vi "Controle_Manip_Main_GUI_WorkingBackup_211222.vi"() -> ()   [LabVIEW 2019] (continued)
            n3621 = call "Shutter.vi"("KCube Shutter Device Reference 2"=w4454, "Shutter Ctrls 2"=w4455, "Shutter on?"=w4453) -> ()
          }
          event "Shutter Mode": Value Change {
            n3622 = event-data() -> ()  [unwired: 1 in, 6 out]
            n3623 = local read "KCube Shutter On?"() -> (w4456:bool)
            n3624 = case shown="True" w4456 {
              frame False {
              }
              frame True {
                # "1 Active == Laser on / Shutter off\n2 Inactive == Laser off / Shutter on\n\nThere are 4 operating modes for shutter:\n1 Manual\n2 Single Toggle\n3 Automatic Toggle\n4 Triggered"
                n3625 = local read "KCube Shutter Device Reference"() -> (w4458:refnum<k24>)
                n3626 = local read "Shutter Mode"() -> (w4457:i32)
                n3627 = invoke class="KCubeSolenoid" method="SetOperatingMode"(reference=w4458, "mode"=w4457) -> ()  [unwired: 2 in, 4 out]
              }
            }
          }
          event "Stop Everything & Quit?": Value Change {
            # "Stop program"
            n3628 = event-data() -> ("NewVal"=w4459:bool)  [unwired: 1 in, 5 out]
            "NewVal" <- w4459
          }
          event "TEC Output", "TEC Temperature", "Laser on? Control": Mouse Down; "Laser Diode Current Set": Value Change {
            # "Laser diode control"
            n3629 = event-data() -> ("CtlRef"=w4461:refnum<vi>)  [unwired: 1 in, 3 out]
            n3630 = local read "Laser Comm On?"() -> (w4460:bool)
            n3631 = case shown="True" w4460 {
              tunnel: w4461 -> [_ w4471]
              frame False {
              }
              frame True {
                n3632 = local read "Photodiode error out"() -> (w4470:errorcluster)
                n3633 = local read "Diode Driver Error"() -> (w4466:errorcluster)
                n3634 = local read "Photodiode handle out"() -> (w4469:refnum<visa-resource-name>)
                n3635 = property class="Ctl"(reference=w4471) -> ("Label.Text"=w4462:string)  [unwired: 1 in, 2 out]
                n3636 = local read "DDE"() -> (w4464:refnum<visa-resource-name>)
                n3637 = case shown="\"Laser on? Control\"" w4462 {
                  tunnel: w4464 -> [w4477 w4488 w4524 w4561 w4594]
                  tunnel: [w4476 w4487 w4523 w4563 w4594] -> w4467
                  tunnel: w4469 -> [w4474 w4483 w4522 w4564 w4593]
                  tunnel: w4470 -> [w4475 w4482 w4521 w4565 w4592]
                  tunnel: [w4474 w4479 w4520 w4564 w4593] -> w4468
                  tunnel: [w4475 w4484 w4519 w4565 w4592] -> w4463
                  tunnel: [w4473 w4481 w4518 w4562 w4591] -> w4465
                  tunnel: w4466 -> [w4472 w4480 w4517 w4560 w4591]
                  frame "TEC Temperature" {
                    n3638 = call <instrlib>:"TL4000 Measure Temperature.vi"("error in (no error)"=w4472, "instrument handle"=w4477) -> ("error out"=w4473:errorcluster, "Temperature"=w4478:dbl, "instrument handle out"=w4476:refnum<visa-resource-name>)  [unwired: 7 in]
                    n3639 = local write "TEC Temperature"(w4478) -> ()
                  }
                  frame "Laser on? Control" {
                    n3640 = flat-sequence {
                      tunnel: w4488 -> [w4496]
                      tunnel: [w4495] -> w4486
                      tunnel: [w4494] -> w4485
                      tunnel: w4480 -> [w4489]
                      tunnel: [w4507] -> w4487
                      tunnel: [w4508] -> w4481
                      tunnel: w4486 -> [w4508]
                      tunnel: w4485 -> [w4507]
                      tunnel: [w4506] -> w4479
                      tunnel: [w4505] -> w4484
                      tunnel: w4483 -> [w4504]
                      tunnel: w4482 -> [w4503]
                      frame #0 {
                        n3641 = call <instrlib>:"TL4000 Get LD Output State.vi"("error in (no error)"=w4489, "instrument handle"=w4496) -> ("error out"=w4491:errorcluster, "LD Output"=w4493:bool, "instrument handle out"=w4492:refnum<visa-resource-name>)  [unwired: 7 in]
                        n3642 = Not(x=w4493) -> (.not. x?=w4490:bool)
                        n3643 = case shown="True" w4490 {
                          selector: w4490 -> [w4498 w4499]
                          frame False {
                            n3644 = Not(x=w4498) -> (.not. x?=w4497:bool)
                            n3645 = property on="TEC Output" class="Bool (strict)"("Visible"=w4497) -> ()  [unwired: 2 in, 2 out]
                          }
                          frame True {
                            n3646 = property on="TEC Output" class="Bool (strict)"("Visible"=w4499) -> ()  [unwired: 2 in, 2 out]
                          }
                        }
                        n3647 = property on="Laser Diode Current Set" class="Slide (strict)"("Visible"=w4490) -> ()  [unwired: 2 in, 2 out]
                        n3648 = property on="Laser Safety" class="Ring (strict)"("Visible"=w4490) -> ()  [unwired: 2 in, 2 out]
                        n3649 = local write "Laser on?"(w4490) -> ()
                        n3650 = call <instrlib>:"TL4000 Switch LD Output.vi"("error in (no error)"=w4491, "LD Output (Off)"=w4490, "instrument handle"=w4492) -> ("error out"=w4495:errorcluster, "instrument handle out"=w4494:refnum<visa-resource-name>)  [unwired: 7 in]
                      }
                      frame #1 {
                        n3651 = local read "PM16-120 On?"() -> (w4500:bool)
                        n3652 = case shown="True" w4500 {
                          tunnel: [w4509 w4516] -> w4506
                          tunnel: [w4510 w4515] -> w4505
                          tunnel: w4504 -> [w4509 w4514]
                          tunnel: w4503 -> [w4510 w4513]
                          tunnel: [0.0 ("Power") w4512] -> w4502
                          frame False {
                          }
                          frame True {
                            n3653 = call <instrlib>:"TLPM Measure Power.vi"("error in (no error)"=w4513, "instrument handle"=w4514) -> ("error out"=w4515:errorcluster, "Power"=w4512:dbl, "instrument handle out"=w4516:refnum<visa-resource-name>)  [unwired: 7 in]
                          }
                        }
                        n3654 = local write "Excitation Power (uW)"(w4502) -> ()
                        n3655 = property on="Excitation Source" class="Enum (strict)"("Val(Sgnl)"=enum16{"P", "CW", "SK"}."CW" ("Value (Signaling)")) -> ()  [unwired: 2 in, 2 out]
                      }
                    }
                  }
                  frame "Laser Diode Current Set" {
                    n3656 = stacked-sequence {
                      seq-local: [w4529 _ _ _] -> [_ _ w4549 _]
                      seq-local: [w4528 _ _ _] -> [_ _ w4548 _]
                      tunnel: w4524 -> [w4533 _ _ _]
                      tunnel: w4517 -> [w4525 _ _ _]
                      tunnel: [_ _ w4549 _] -> w4523
                      tunnel: [_ _ w4548 _] -> w4518
                      tunnel: w4522 -> [_ _ w4547 _]
                      tunnel: w4521 -> [_ _ w4546 _]
                      tunnel: [_ _ w4545 _] -> w4520
                      tunnel: [_ _ w4544 _] -> w4519
                      frame #0 {
                        n3657 = local read "Laser Diode Current Set"() -> (w4526:dbl)
                        n3658 = call <instrlib>:"TL4000 Get Laser Diode Current Setpoint.vi"("error in (no error)"=w4525, "instrument handle"=w4533) -> ("error out"=w4530:errorcluster, "Laser Diode Current Setpoint"=w4532:dbl, "instrument handle out"=w4531:refnum<visa-resource-name>)  [unwired: 7 in]
                        n3659 = Not Equal?(x=w4526, y=w4532) -> (x != y?=w4527:bool)
                        n3660 = case shown="True" w4527 {
                          tunnel: w4531 -> [w4535 w4540]
                          tunnel: w4530 -> [w4534 w4539]
                          tunnel: [w4535 w4538] -> w4529
                          tunnel: [w4534 w4537] -> w4528
                          tunnel: w4526 -> [_ w4536]
                          frame False {
                          }
                          frame True {
                            n3661 = call <instrlib>:"TL4000 Set Laser Diode Current Setpoint.vi"("error in (no error)"=w4539, "Laser Diode Current Setpoint (0.0)"=w4536, "instrument handle"=w4540) -> ("error out"=w4537:errorcluster, "instrument handle out"=w4538:refnum<visa-resource-name>)  [unwired: 7 in]
                          }
                        }
                      }
                      frame #1 {
                        n3662 = Wait (ms)(milliseconds to wait=u32 50) -> ()  [unwired: 1 out]
                      }
                      frame #2 {
                        n3663 = local read "PM16-120 On?"() -> (w4542:bool)
                        n3664 = case shown="True" w4542 {
                          tunnel: w4547 -> [w4552 w4557]
                          tunnel: w4546 -> [w4551 w4556]
                          tunnel: [w4552 w4555] -> w4545
                          tunnel: [w4551 w4554] -> w4544
                          tunnel: [0.0 ("Power") w4553] -> w4543
                          frame False {
                          }
                          frame True {
                            n3665 = call <instrlib>:"TLPM Measure Power.vi"("error in (no error)"=w4556, "instrument handle"=w4557) -> ("error out"=w4554:errorcluster, "Power"=w4553:dbl, "instrument handle out"=w4555:refnum<visa-resource-name>)  [unwired: 7 in]
                          }
                        }
                        n3666 = local write "Excitation Power (uW)"(w4543) -> ()
                      }
                      frame #3 {
                        n3667 = local write "Background taken?"(FALSE ("Background taken?")) -> ()
                      }
                    }
                  }
                  frame "TEC Output" {
                    n3668 = local read "TEC Output"() -> (w4559:bool)
                    n3669 = call <instrlib>:"TL4000 Switch TEC Output.vi"("error in (no error)"=w4560, "TEC Output (Off)"=w4559, "instrument handle"=w4561) -> ("error out"=w4566:errorcluster, "instrument handle out"=w4567:refnum<visa-resource-name>)  [unwired: 7 in]
                    n3670 = case shown="True" w4559 {
                      tunnel: w4567 -> [w4569 w4576]
                      tunnel: w4566 -> [w4568 w4575]
                      tunnel: [w4569 w4572] -> w4563
                      tunnel: [w4568 w4571] -> w4562
                      frame False {
                      }
                      frame True {
                        n3671 = while {
                          tunnel: w4576 -> [w4590]
                          tunnel: [w4582] -> w4573
                          tunnel: w4575 -> [w4589]
                          tunnel: [w4583] -> w4574
                          stop <- w4577 stop-if-true
                          n3672 = call <instrlib>:"TL4000 Measure Temperature.vi"("error in (no error)"=w4589, "instrument handle"=w4590) -> ("error out"=w4583:errorcluster, "Temperature"=w4580:dbl, "instrument handle out"=w4582:refnum<visa-resource-name>)  [unwired: 7 in]
                          n3673 = Wait (ms)(milliseconds to wait=u32 250) -> ()  [unwired: 1 out]
                          n3674 = local write "TEC Temperature"(w4580) -> ()
                          n3675 = Subtract(x=w4580, y=25.0) -> (x-y=w4587:dbl)
                          n3676 = Absolute Value(x=w4587) -> (abs(x)=w4586:dbl)
                          n3677 = Equal?(x=w4580, y=0.0) -> (x = y?=w4578:bool)
                          n3678 = Less?(x=w4586, y=0.01) -> (x < y?=w4581:bool)
                          n3679 = Or(x=w4581, y=w4578) -> (x .or. y?=w4577:bool)
                        }
                        n3680 = call <instrlib>:"TL4000 Measure Temperature.vi"("error in (no error)"=w4574, "instrument handle"=w4573) -> ("error out"=w4571:errorcluster, "Temperature"=w4570:dbl, "instrument handle out"=w4572:refnum<visa-resource-name>)  [unwired: 7 in]
                        n3681 = local write "TEC Temperature"(w4570) -> ()
                      }
                    }
                    n3682 = property on="Laser on? Control" class="Bool (strict)"("Visible"=w4559) -> ()  [unwired: 2 in, 2 out]
                  }
                  frame Default {
                  }
                }
                "Diode Driver Error out" <- w4465
                n3683 = local write "Photodiode error out"(w4463) -> ()
                n3684 = local write "Photodiode handle out"(w4468) -> ()
                n3685 = local write "Diode Driver COM"(w4467) -> ()
              }
            }
          }
          event "Fit?": Mouse Down {
            n3686 = event-data() -> ()  [unwired: 1 in, 8 out]
            n3687 = property on="CCD 1D Spectrum Main" class="XYGraph (strict)"() -> ("Value"=w4599:cluster{dbl[], dbl[]})  [unwired: 2 in, 2 out]
            n3688 = local read "BackgroundSpec"() -> (w4595:dbl[])
            n3689 = Unbundle(w4599) -> (w4598:dbl[], w4596:dbl[])
            n3690 = call "subVI_FitLorentzien.vi"("Background Spec"=w4595, "X"=w4598, "Y"=w4596) -> ("best fit parameters"=→"best fit parameters":dbl[])  [unwired: 1 in, 3 out]
          }
          event "Temperature (K)": Mouse Down {
            n3691 = event-data() -> ()  [unwired: 1 in, 8 out]
            n3692 = local read "Cryostation On?"() -> (w4600:bool)
            n3693 = case shown="True" w4600 {
              frame False {
              }
              frame True {
                w4602 = 10.0 ("y")
                n3694 = local read "Cryostation ID"() -> (w4612:refnum<k5>)
                n3695 = call "GetCryoInfo.vi"("connection ID"=w4612) -> ("User Stability"=w4607:dbl, "User Temp"=w4608:dbl, "connection ID out"=w4606:refnum<k5>, "Sample Stability"=w4609:dbl, "Sample Temp"=w4605:dbl, "Platform Stability"=w4610:dbl, "Platform Temp"=w4611:dbl)  [unwired: 4 in]
                n3696 = local write "Cryo Platform Temp"(w4611) -> ()
                n3697 = Multiply(x=w4605, y=w4602) -> (x*y=w4604:dbl)
                n3698 = local write "Cryo Sample Stability"(w4609) -> ()
                n3699 = local write "Cryostation ID"(w4606) -> ()
                n3700 = local write "Cryo User Stability"(w4607) -> ()
                n3701 = local write "Cryo Sample Temp"(w4605) -> ()
                n3702 = local write "Cryo Platform Stability"(w4610) -> ()
                n3703 = local write "Cryo User Temp"(w4608) -> ()
                n3704 = Round To Nearest(number=w4604) -> (nearest integer value=w4603:dbl)
                n3705 = Divide(x=w4603, y=w4602) -> (x/y=w4601:dbl)
                n3706 = local write "Temperature (K)"(w4601) -> ()
              }
            }
          }
          event "Voltage Output?": Value Change {
            w4617 = u8 2 items=["1", "2", "3"] ("axis")
            w4618 = u8 1 items=["1", "2", "3"] ("axis")
            w4619 = u8 0 items=["1", "2", "3"] ("axis")
            n3707 = event-data() -> ("NewVal"=w4613:bool)  [unwired: 1 in, 5 out]
            n3708 = local read "Att DeviceHandle"() -> (w4628:u64)
            n3709 = local read "Att Error"() -> (w4626:errorcluster)
            n3710 = local read "ourDLL"() -> (w4616:path)
            n3711 = call "ANC350v4_SetAxisOutput.vi"("deviceHandle"=w4628, "Path to *.DLL"=w4616, "axis"=w4619, "enable"=w4613, "autoDisable"=TRUE, "error in"=w4626) -> ("deviceHandle"=w4624:u64, "error ANC350v4_setAxisOutput"=w4625:errorcluster)  [unwired: 7 in, 1 out]
            n3712 = call "ANC350v4_SetAxisOutput.vi"("deviceHandle"=w4624, "Path to *.DLL"=w4616, "axis"=w4618, "enable"=w4613, "autoDisable"=TRUE, "error in"=w4625) -> ("deviceHandle"=w4623:u64, "error ANC350v4_setAxisOutput"=w4622:errorcluster)  [unwired: 7 in, 1 out]
            n3713 = call "ANC350v4_SetAxisOutput.vi"("deviceHandle"=w4623, "Path to *.DLL"=w4616, "axis"=w4617, "enable"=w4613, "autoDisable"=TRUE, "error in"=w4622) -> ("deviceHandle"=w4615:u64, "error ANC350v4_setAxisOutput"=w4614:errorcluster)  [unwired: 7 in, 1 out]
            n3714 = local write "Att Error"(w4614) -> ()
            n3715 = local write "Att DeviceHandle"(w4615) -> ()
          }
          event Timeout {
            # "Use timeout case to send data to globals"
            n3716 = event-data() -> ()  [unwired: 1 in, 3 out]
          }
        }
      }
      n3717 = while {
        stop <- w696 stop-if-true
        # "Separate loop for \"measurements\" requiring simultaneous optimisation of experimental parameters: continuous modes"
        n3718 = event shown="[2] \"Acquire PD\": Mouse Down" {
          selector: _ -> [_ _ _]
          dyn-events: _ -> [_ _ _]
          timeout: 500 -> [_ _ _]
          event Timeout {
            n3719 = event-data() -> ()  [unwired: 1 in, 3 out]
          }
          event "Fast Acq Continuous": Mouse Down {
            n3720 = event-data() -> ()  [unwired: 1 in, 8 out]
            n3721 = local read "Acq Mode"() -> (w697:T3)
            n3722 = case shown="\"Spectrum\", Default" w697 {
              frame "Image" {
              }
              frame "APD 1" {
              }
              frame "Spectrum", Default {
                n3723 = stacked-sequence {
                  frame #0 {
                    # "prep stuff"
                    n3724 = property on="Experiment Graph Controls" class="TabCtl (strict)"("Value"=T25."Spectrum" ("Experiment Graph Controls")) -> ()  [unwired: 2 in, 2 out]
                  }
                  frame #1 {
                    # "open shutter once"
                    n3725 = control-ref of="Shutter Ctrls"() -> (w704:refnum<vi>)
                    n3726 = local read "KCube Shutter On?"() -> (w701:bool)
                    n3727 = local read "Acq Mode"() -> (w702:T3)
                    n3728 = control-ref of="KCube Shutter Device Reference"() -> (w703:refnum<vi>)
                    n3729 = call "Shutter.vi"("KCube Shutter Device Reference 2"=w703, "Shutter Ctrls 2"=w704, "Shutter on?"=w701) -> ()
                    n3730 = case shown="\"Spectrum\", Default" w702 {
                      frame "Spectrum", Default {
                        n3731 = property on="CCD 1D Spectrum Main" class="XYGraph (strict)"("Visible"=TRUE) -> ()  [unwired: 2 in, 2 out]
                        n3732 = property on="CCD 2D Image Main" class="IntGraph (strict)"("Visible"=FALSE) -> ()  [unwired: 2 in, 2 out]
                      }
                      frame "Image" {
                        n3733 = property on="CCD 1D Spectrum Main" class="XYGraph (strict)"("Visible"=FALSE) -> ()  [unwired: 2 in, 2 out]
                        n3734 = property on="CCD 2D Image Main" class="IntGraph (strict)"("Visible"=TRUE) -> ()  [unwired: 2 in, 2 out]
                      }
                    }
                    n3735 = control-ref of="MasterStop"() -> (w700:refnum<vi>)
                    n3736 = property class="Bool (strict)"(reference=w700, "Visible"=TRUE) -> ()  [unwired: 1 in, 2 out]
                  }
                  frame #2 {
                    # "acquire 1000 spectra"
                    n3737 = for {
                      N: 1000 -> [_]
                      stop <- w724 stop-if-true
                      n3738 = local read "CCD ROI"() -> (w719:T20)
                      n3739 = local read "LightField Automation out"() -> (w723:refnum<class "LightField Automation.lvclass">)
                      n3740 = local read "Acq Mode"() -> (w726:T3)
                      n3741 = local read "LightField Automation error out"() -> (w720:errorcluster)
                      n3742 = local read "Accumulations"() -> (w727:dbl)
                      n3743 = control-ref of="MasterStop"() -> (w710:refnum<vi>)
                      n3744 = local read "BackgroundSpec"() -> (w712:dbl[])
                      n3745 = local read "Excitation Power (uW)"() -> (w715:dbl)
                      n3746 = call "LFA_Capture.vi"("error in (no error)"=w720, "Frames"=w727, "LightField Automation in"=w723) -> ("error out"=w721:errorcluster, "Data"=w725:T26, "LightField Automation out"=w722:refnum<class "LightField Automation.lvclass">)  [unwired: 6 in]
                      n3747 = case shown="\"Spectrum\", Default" w726 {
                        selector: w726 -> [w735 w741]
                        tunnel: w725 -> [w736 w743]
                        tunnel: w719 -> [w732 w738]
                        tunnel: [w728 w737] -> w716
                        frame "Spectrum", Default {
                          n3748 = local read "Wavelength calibration"() -> (w730:dbl[])
                          n3749 = Divide(x=1239.842, y=w730) -> (x/y=w729:dbl[])
                          n3750 = call "PrepareData4Graph.vi"("Wavelength nm"=w729, "DataLF"=w736, "CCD ROI"=w732, "AcqMode"=w735, "Data type"=T30."Spectre") -> ("Spectrum"=w734:cluster{"Array 2":dbl[], "Array":dbl[]}, "PLInt out"=w728:dbl[])  [unwired: 2 in, 2 out]
                          n3751 = local write "CCD 1D Spectrum Main"(w734) -> ()
                        }
                        frame "Image" {
                          n3752 = local read "Wavelength calibration"() -> (w742:dbl[])
                          n3753 = call "PrepareData4Graph.vi"("Wavelength nm"=w742, "DataLF"=w743, "CCD ROI"=w738, "AcqMode"=w741, "Data type"=T30."Spectre") -> ("Intensity Graph"=w740:dbl[][], "PLInt out"=w737:dbl[])  [unwired: 2 in, 2 out]
                          n3754 = local write "CCD 2D Image Main"(w740) -> ()
                        }
                      }
                      n3755 = call "myMax.vi"("Array"=w716) -> ("myMax"=w718:dbl)  [unwired: 1 in]
                      n3756 = property on="CCD 1D Spectrum Main" class="XYGraph (strict)"("YScale.Maximum"=w718, "YScale.Minimum"=0.0 ("Y Scale.Range:Minimum")) -> ()  [unwired: 2 in, 2 out]
                      n3757 = local read "Acq Time (ms)"() -> (w714:dbl)
                      n3758 = local read "Display Mode"() -> (w711:u16)
                      n3759 = local write "LightField Automation out"(w722) -> ()
                      n3760 = local write "LightField Automation error out"(w721) -> ()
                      n3761 = property class="Bool (strict)"(reference=w710) -> ("Value"=w724:bool)  [unwired: 1 in, 2 out]
                      n3762 = control-ref of="Cnts"() -> (w713:refnum<vi>)
                      n3763 = call "2Cnts.vi"("Array Background"=w712, "Pow W"=w715, "AcqTime ms"=w714, "Cnts Ref"=w713, "Display Mode"=w711, "Array"=w716) -> ()  [unwired: 1 out]
                    }
                  }
                  frame #3 {
                    # "close shutter"
                    n3764 = local read "KCube Shutter On?"() -> (w747:bool)
                    n3765 = control-ref of="Fast Acq Continuous"() -> (w745:refnum<vi>)
                    n3766 = control-ref of="Shutter Ctrls"() -> (w751:refnum<vi>)
                    n3767 = control-ref of="KCube Shutter Device Reference"() -> (w750:refnum<vi>)
                    n3768 = control-ref of="MasterStop"() -> (w746:refnum<vi>)
                    n3769 = property class="Bool (strict)"(reference=w745, "Value"=FALSE) -> ()  [unwired: 1 in, 2 out]
                    n3770 = call "Shutter.vi"("KCube Shutter Device Reference 2"=w750, "Shutter Ctrls 2"=w751, "Shutter on?"=w747) -> ()
                    n3771 = property class="Bool (strict)"(reference=w746, "Value"=FALSE, "Visible"=FALSE) -> ()  [unwired: 1 in, 2 out]
                  }
                }
              }
            }
          }
          event "Acquire PD": Mouse Down {
            n3772 = event-data() -> ()  [unwired: 1 in, 8 out]
            n3773 = local read "PicoHarp On?"() -> (w752:bool)
            n3774 = case shown="True" w752 {
              frame False {
              }
              frame True {
                n3775 = local read "Spectrum Custom Continuous Mode"() -> (w753:u16)
                n3776 = case shown="3" w753 {
                  frame 0, Default {
                    # "PD 2"
                    n3777 = stacked-sequence {
                      frame #0 {
                        n3778 = property on="Experiment Graph Controls" class="TabCtl (strict)"("Value"=T25."APDs" ("Experiment Graph Controls")) -> ()  [unwired: 2 in, 2 out]
                      }
                      frame #1 {
                        n3779 = for {
                          N: 1000 -> [_]
                          shift-right: [w759] -> _
                          shift-left: dbl[] [] -> [w764]
                          stop <- w757 stop-if-true
                          n3780 = local read "Photodiode handle out"() -> (w770:refnum<visa-resource-name>)
                          n3781 = local read "Photodiode error out"() -> (w769:errorcluster)
                          n3782 = control-ref of="PD 1D Spectrum"() -> (w761:refnum<vi>)
                          n3783 = Tick Count (ms)() -> (millisecond timer value=w766:u32)
                          n3784 = while {
                            shift-right: [w780] -> w768
                            shift-left: w770 -> [w783]
                            shift-right: [w779] -> w767
                            shift-left: w769 -> [w782]
                            tunnel: w766 -> [w776]
                            shift-right: [w771] -> w763
                            shift-left: dbl[] [] -> [w773]
                            stop <- w775 stop-if-true
                            n3785 = local read "Acq Time (ms)"() -> (w774:dbl)
                            n3786 = Tick Count (ms)() -> (millisecond timer value=w778:u32)
                            n3787 = call <instrlib>:"TLPM Measure Power.vi"("error in (no error)"=w782, "instrument handle"=w783) -> ("error out"=w779:errorcluster, "Power"=w772:dbl, "instrument handle out"=w780:refnum<visa-resource-name>)  [unwired: 7 in]
                            n3788 = control-ref of="Excitation Power (uW)"() -> (w781:refnum<vi>)
                            n3789 = property class="DigNum (strict)"(reference=w781, "Value"=w772) -> ()  [unwired: 1 in, 2 out]
                            n3790 = Subtract(x=w778, y=w776) -> (x-y=w777:u32)
                            n3791 = Insert Into Array(array=w773, new element=w772) -> (w771:dbl[])  [unwired: 1 in]
                            n3792 = Greater?(x=w777, y=w774) -> (0:w775:bool)
                          }
                          n3793 = control-ref of="Stop PD"() -> (w758:refnum<vi>)
                          n3794 = local write "Photodiode handle out"(w768) -> ()
                          n3795 = call-poly <vilib>:"Mean.vi"("X"=w763) -> ("mean"=w762:dbl)  [unwired: 1 out]
                          n3796 = Insert Into Array(array=w764, new element=w762) -> (w759:dbl[])  [unwired: 1 in]
                          n3797 = Build Array(w759) -> (w760:dbl[][])
                          n3798 = property class="WFGraph (strict)"(reference=w761, "Value"=w760) -> ()  [unwired: 1 in, 2 out]
                          n3799 = local write "Photodiode error out"(w767) -> ()
                          n3800 = property class="Bool (strict)"(reference=w758) -> ("Value"=w757:bool)  [unwired: 1 in, 2 out]
                        }
                      }
                      frame #2 {
                        w784 = FALSE ("Stop PD")
                        n3801 = property on="Acquire PD" class="Bool (strict)"("Value"=w784) -> ()  [unwired: 2 in, 2 out]
                        n3802 = property on="Stop PD" class="Bool (strict)"("Value"=w784) -> ()  [unwired: 2 in, 2 out]
                      }
                    }
                  }
                  frame 3 {
                    # "APD1+2"
                    n3803 = stacked-sequence {
                      frame #0 {
                        n3804 = local read "PH_Init_Data"() -> (w797:T11)
                        n3805 = Unbundle By Name(w797) -> ("Deviceindex"=w789:i32)
                        n3806 = local read "PH_Settings_Params"() -> (w790:T10)
                        n3807 = local read "PH_CFD1 level"() -> (w794:i32)
                        n3808 = local read "PH_CFD1 zero X"() -> (w793:i32)
                        n3809 = local read "Acq Time (ms)"() -> (w792:dbl)
                        n3810 = local read "PH_Range No."() -> (w788:i32)
                        n3811 = local read "PH_CFD0 level"() -> (w795:i32)
                        n3812 = local read "PH_CFD0 zero X"() -> (w787:i32)
                        n3813 = local read "PH_SyncDiv"() -> (w796:enum16{"1", "2", "4", "8"})
                        n3814 = property on="Experiment Graph Controls" class="TabCtl (strict)"("Value"=T25."APDs" ("Experiment Graph Controls")) -> ()  [unwired: 2 in, 2 out]
                        n3815 = Bundle By Name(cluster=w790, "SyncDiv"=w796, "DeviceIndex"=w789, "CFD0 level"=w795, "CFD0 zero X"=w787, "CFD1 level"=w794, "CFD1 zero X"=w793, "Range No."=w788, "StopOnOverflow"=TRUE, "AcqTime (ms)"=w792) -> (w785:T10)
                        n3816 = local write "PH_Settings_Params"(w785) -> ()
                      }
                      frame #1 {
                        n3817 = local read "PH_Init_Data"() -> (w800:T11)
                        n3818 = local read "PH_Settings_Params"() -> (w801:T10)
                        n3819 = control-ref of="Stop PD"() -> (w802:refnum<vi>)
                        n3820 = control-ref of="PD 1D Spectrum"() -> (w803:refnum<vi>)
                        n3821 = call "PH_GetRates_SubVI.vi"("APD num"=enum16{"NA", "APD1", "APD2", "APD1+2"}."APD1+2", "PH_Settings_Params"=w801, "PH_Init_Data"=w800, "Stop PD Ref"=w802, "PD 1D Spectrum Ref"=w803) -> ("APD1+2"=w798:dbl[][])  [unwired: 6 in]
                        n3822 = local write "PD Data 2D 2"(w798) -> ()
                      }
                      frame #2 {
                        w804 = FALSE ("Stop PD")
                        n3823 = property on="Acquire PD" class="Bool (strict)"("Value"=w804) -> ()  [unwired: 2 in, 2 out]
                        n3824 = property on="Stop PD" class="Bool (strict)"("Value"=w804) -> ()  [unwired: 2 in, 2 out]
                      }
                    }
                  }
                  frame 1 {
                    # "APD1"
                    n3825 = stacked-sequence {
                      frame #0 {
                        n3826 = local read "PH_Init_Data"() -> (w817:T11)
                        n3827 = Unbundle By Name(w817) -> ("Deviceindex"=w809:i32)
                        n3828 = local read "PH_Settings_Params"() -> (w810:T10)
                        n3829 = local read "PH_CFD1 level"() -> (w814:i32)
                        n3830 = local read "PH_CFD1 zero X"() -> (w813:i32)
                        n3831 = local read "Acq Time (ms)"() -> (w812:dbl)
                        n3832 = local read "PH_Range No."() -> (w808:i32)
                        n3833 = local read "PH_CFD0 level"() -> (w815:i32)
                        n3834 = local read "PH_CFD0 zero X"() -> (w807:i32)
                        n3835 = local read "PH_SyncDiv"() -> (w816:enum16{"1", "2", "4", "8"})
                        n3836 = property on="Experiment Graph Controls" class="TabCtl (strict)"("Value"=T25."APDs" ("Experiment Graph Controls")) -> ()  [unwired: 2 in, 2 out]
                        n3837 = Bundle By Name(cluster=w810, "SyncDiv"=w816, "DeviceIndex"=w809, "CFD0 level"=w815, "CFD0 zero X"=w807, "CFD1 level"=w814, "CFD1 zero X"=w813, "Range No."=w808, "StopOnOverflow"=TRUE, "AcqTime (ms)"=w812) -> (w805:T10)
                        n3838 = local write "PH_Settings_Params"(w805) -> ()
                      }
                      frame #1 {
                        n3839 = local read "PH_Init_Data"() -> (w820:T11)
                        n3840 = local read "PH_Settings_Params"() -> (w821:T10)
                        n3841 = control-ref of="Stop PD"() -> (w822:refnum<vi>)
                        n3842 = control-ref of="PD 1D Spectrum"() -> (w823:refnum<vi>)
                        n3843 = call "PH_GetRates_SubVI.vi"("APD num"=enum16{"NA", "APD1", "APD2", "APD1+2"}."APD1", "PH_Settings_Params"=w821, "PH_Init_Data"=w820, "Stop PD Ref"=w822, "PD 1D Spectrum Ref"=w823) -> ("APD1+2"=w818:dbl[][])  [unwired: 6 in]
                        n3844 = local write "PD Data 2D 2"(w818) -> ()
                      }
                      frame #2 {
                        w824 = FALSE ("Stop PD")
                        n3845 = property on="Acquire PD" class="Bool (strict)"("Value"=w824) -> ()  [unwired: 2 in, 2 out]
                        n3846 = property on="Stop PD" class="Bool (strict)"("Value"=w824) -> ()  [unwired: 2 in, 2 out]
                      }
                    }
                  }
                  frame 2 {
                    # "APD2"
                    n3847 = stacked-sequence {
                      frame #0 {
                        n3848 = local read "PH_Init_Data"() -> (w837:T11)
                        n3849 = Unbundle By Name(w837) -> ("Deviceindex"=w829:i32)
                        n3850 = local read "PH_Settings_Params"() -> (w830:T10)
                        n3851 = local read "PH_CFD1 level"() -> (w834:i32)
                        n3852 = local read "PH_CFD1 zero X"() -> (w833:i32)
                        n3853 = local read "Acq Time (ms)"() -> (w832:dbl)
                        n3854 = local read "PH_Range No."() -> (w828:i32)
                        n3855 = local read "PH_CFD0 level"() -> (w835:i32)
                        n3856 = local read "PH_CFD0 zero X"() -> (w827:i32)
                        n3857 = local read "PH_SyncDiv"() -> (w836:enum16{"1", "2", "4", "8"})
                        n3858 = property on="Experiment Graph Controls" class="TabCtl (strict)"("Value"=T25."APDs" ("Experiment Graph Controls")) -> ()  [unwired: 2 in, 2 out]
                        n3859 = Bundle By Name(cluster=w830, "SyncDiv"=w836, "DeviceIndex"=w829, "CFD0 level"=w835, "CFD0 zero X"=w827, "CFD1 level"=w834, "CFD1 zero X"=w833, "Range No."=w828, "StopOnOverflow"=TRUE, "AcqTime (ms)"=w832) -> (w825:T10)
                        n3860 = local write "PH_Settings_Params"(w825) -> ()
                      }
                      frame #1 {
                        n3861 = local read "PH_Init_Data"() -> (w840:T11)
                        n3862 = local read "PH_Settings_Params"() -> (w841:T10)
                        n3863 = control-ref of="Stop PD"() -> (w842:refnum<vi>)
                        n3864 = control-ref of="PD 1D Spectrum"() -> (w843:refnum<vi>)
                        n3865 = call "PH_GetRates_SubVI.vi"("APD num"=enum16{"NA", "APD1", "APD2", "APD1+2"}."APD2", "PH_Settings_Params"=w841, "PH_Init_Data"=w840, "Stop PD Ref"=w842, "PD 1D Spectrum Ref"=w843) -> ("APD1+2"=w838:dbl[][])  [unwired: 6 in]
                        n3866 = local write "PD Data 2D 2"(w838) -> ()
                      }
                      frame #2 {
                        w844 = FALSE ("Stop PD")
                        n3867 = property on="Acquire PD" class="Bool (strict)"("Value"=w844) -> ()  [unwired: 2 in, 2 out]
                        n3868 = property on="Stop PD" class="Bool (strict)"("Value"=w844) -> ()  [unwired: 2 in, 2 out]
                      }
                    }
                  }
                }
              }
            }
          }
        }
        n3869 = local read "NewVal"() -> (w696:bool)
      }
    }
    frame #3 {
      # "Shutdown: close all open references and connections"
      n3870 = stacked-sequence {
        frame #0 {
          # "Is the sample to be kept and reused?\ni.e. does LabVIEW keep sample details or empty them"
          n3871 = Two Button Dialog(message="Do you want to keep the sample details in LV?", 1:"No thanks." ("F button name (\"Cancel\")"), 2:"Yes please!" ("T button name (\"OK\")")) -> (T button?=w4629:bool)
          n3872 = case shown="False" w4629 {
            frame False {
              n3873 = local write "SampleGoal"("") -> ()
            }
            frame True {
            }
          }
        }
        frame #1 {
          # "Shutdown all connections"
          n3874 = local read "Initialise all devices?"() -> (w4634:bool)
          n3875 = case shown="True" w4634 {
            frame False {
              # "No devices to deactivate"
            }
            frame True {
              # "Deactivate all the selected devices"
              n3876 = stacked-sequence {
                frame #0 {
                  # "Message to user"
                  n3877 = local read "Log file"() -> (w4638:string)
                  n3878 = call "Write2LogFile.vi"("Add to log file"="Closing all connections ...", "Log file before"=w4638, "Checkbox"=FALSE) -> ("Log file after"=w4637:string)
                  n3879 = local write "Log file"(w4637) -> ()
                }
                frame #1 {
                  # "LLTF"
                  n3880 = local read "LLTF On?"() -> (w4639:bool)
                  n3881 = case shown="True" w4639 {
                    frame False {
                    }
                    frame True {
                      n3882 = local read "LLTF Reference"() -> (w4641:refnum<k7>)
                      n3883 = local read "LLTF Error"() -> (w4640:errorcluster)
                      n3884 = Close Reference(reference=w4641, error in (no error)=w4640) -> ()  [unwired: 1 out]
                    }
                  }
                }
                frame #2 {
                  # "turn off laser output, TEC and close connection"
                  # "448.3nm Laser Diode + Temp Controller & Driver"
                  n3885 = local read "Laser Comm On?"() -> (w4642:bool)
                  n3886 = case shown="True" w4642 {
                    frame False {
                      w4643 = TRUE ("Visible")
                      n3887 = property on="TEC Output" class="Bool (strict)"("Visible"=w4643) -> ()  [unwired: 2 in, 2 out]
                      n3888 = property on="TEC Temperature" class="DigNum (strict)"("Visible"=w4643) -> ()  [unwired: 2 in, 2 out]
                    }
                    frame True {
                      w4645 = FALSE ("TEC Output (Off)")
                      w4644 = FALSE ("LD Output (Off)")
                      # "laser"
                      n3889 = local read "Diode Driver COM"() -> (w4647:refnum<visa-resource-name>)
                      n3890 = local read "Diode Driver Error"() -> (w4646:errorcluster)
                      n3891 = property on="Laser on? Control" class="Bool (strict)"("Visible"=w4644) -> ()  [unwired: 2 in, 2 out]
                      n3892 = Not(x=w4644) -> (.not. x?=w4652:bool)
                      n3893 = call <instrlib>:"TL4000 Switch LD Output.vi"("error in (no error)"=w4646, "LD Output (Off)"=w4644, "instrument handle"=w4647) -> ("error out"=w4648:errorcluster, "instrument handle out"=w4651:refnum<visa-resource-name>)  [unwired: 7 in]
                      n3894 = property on="Laser Safety" class="Ring (strict)"("Visible"=w4644) -> ()  [unwired: 2 in, 2 out]
                      n3895 = local write "Laser on?"(w4644) -> ()
                      n3896 = local write "Laser on? Control"(w4644) -> ()
                      n3897 = property on="TEC Output" class="Bool (strict)"("Visible"=w4652) -> ()  [unwired: 2 in, 2 out]
                      n3898 = call <instrlib>:"TL4000 Switch TEC Output.vi"("error in (no error)"=w4648, "TEC Output (Off)"=w4645, "instrument handle"=w4651) -> ("error out"=w4649:errorcluster, "instrument handle out"=w4650:refnum<visa-resource-name>)  [unwired: 7 in]
                      n3899 = call <instrlib>:"TL4000 Close.vi"("error in (no error)"=w4649, "instrument handle"=w4650) -> ()  [unwired: 9 in, 1 out]
                      n3900 = local write "TEC Output"(w4645) -> ()
                      n3901 = property on="Laser Diode Current Set" class="Slide (strict)"("Visible"=w4644) -> ()  [unwired: 2 in, 2 out]
                      n3902 = property on="TEC Temperature" class="DigNum (strict)"("Visible"=w4652) -> ()  [unwired: 2 in, 2 out]
                    }
                  }
                }
                frame #3 {
                  # "KCubes: 1 Shutter + 3 Piezos"
                  n3903 = local read "KCubes Piezo On?"() -> (w4654:bool)
                  n3904 = case shown="True" w4654 {
                    frame False {
                    }
                    frame True {
                      # "Close piezo controls and shutter device"
                      n3905 = local read "KCubePiezoControl Y Reference"() -> (w4657:refnum<k24>)
                      n3906 = local read "KCubePiezoControl X Reference"() -> (w4656:refnum<k24>)
                      n3907 = local read "KCubePiezoControl Z Reference"() -> (w4658:refnum<k24>)
                      n3908 = invoke class="KCubePiezoControl" method="CloseDevice"(reference=w4657) -> ()  [unwired: 2 in, 3 out]
                      n3909 = invoke class="KCubePiezoControl" method="CloseDevice"(reference=w4656) -> ()  [unwired: 2 in, 3 out]
                      n3910 = invoke class="KCubePiezoControl" method="CloseDevice"(reference=w4658) -> ()  [unwired: 2 in, 3 out]
                    }
                  }
                  n3911 = local read "KCube Shutter On?"() -> (w4653:bool)
                  n3912 = case shown="True" w4653 {
                    frame False {
                    }
                    frame True {
                      n3913 = local read "KCubeSolenoidControl Reference"() -> (w4655:refnum<k24>)
                      n3914 = invoke class="KCubeSolenoidControl" method="CloseDevice"(reference=w4655) -> ()  [unwired: 2 in, 3 out]
                    }
                  }
                }
                frame #4 {
                  # "LightField: SpectraPro Mono + CCD"
                  n3915 = local read "LightField On?"() -> (w4659:bool)
                  n3916 = case shown="True" w4659 {
                    frame False {
                    }
                    frame True {
                      n3917 = local read "LightField Automation error out"() -> (w4660:errorcluster)
                      n3918 = local read "LightField Automation out"() -> (w4661:refnum<class "LightField Automation.lvclass">)
                      n3919 = call "LFA_Close.vi"("error in (no error)"=w4660, "LightField Automation in"=w4661) -> ()  [unwired: 8 in, 2 out]
                    }
                  }
                }
                frame #5 {
                  # "ESP 301: 2 rotation stages + 1 linear translation stage"
                  n3920 = local read "ESP 301 On?"() -> (w4662:bool)
                  n3921 = case shown="True" w4662 {
                    frame False {
                    }
                    frame True {
                      n3922 = local read "ESP 301 COM Port"() -> (w4663:refnum<visa-resource-name>)
                      n3923 = call "Close.vi"("VISA resource name"=w4663) -> ()  [unwired: 10 in, 1 out]
                    }
                  }
                }
                frame #6 {
                  # "ESP 300: Mono Jobin Yvon"
                  n3924 = local read "ESP 300 On?"() -> (w4664:bool)
                  n3925 = case shown="True" w4664 {
                    frame False {
                    }
                    frame True {
                      n3926 = local read "ESP300 COM Port"() -> (w4665:refnum<visa-resource-name>)
                      n3927 = local read "ESP300 Error"() -> (w4666:errorcluster)
                      n3928 = call "Uninit Communication.vi"("error in (no error)"=w4666, "VISA resource name in"=w4665) -> ()  [unwired: 9 in, 1 out]
                    }
                  }
                }
                frame #7 {
                  # "Thorlabs USB photodiode"
                  n3929 = local read "PM16-120 On?"() -> (w4667:bool)
                  n3930 = case shown="True" w4667 {
                    frame False {
                    }
                    frame True {
                      # "photo"
                      n3931 = local read "Photodiode error out"() -> (w4672:errorcluster)
                      n3932 = call <instrlib>:"TLPM Measure Power.vi"("error in (no error)"=w4672, "instrument handle"=refnum<visa-resource-name> "USB0::0x1313::0x807B::190927109::INSTR") -> ("error out"=w4670:errorcluster, "Power"=w4669:dbl, "instrument handle out"=w4671:refnum<visa-resource-name>)  [unwired: 7 in]
                      n3933 = call <instrlib>:"TLPM Close.vi"("error in (no error)"=w4670, "instrument handle"=w4671) -> ("error out"=w4673:errorcluster)  [unwired: 9 in]
                      n3934 = local write "Excitation Power (uW)"(w4669) -> ()
                      n3935 = local write "Photodiode error out"(w4673) -> ()
                    }
                  }
                }
                frame #8 {
                  # "Attocubes disconnect"
                  n3936 = local read "Attocubes On?"() -> (w4674:bool)
                  n3937 = case shown="True" w4674 {
                    frame False {
                    }
                    frame True {
                      w4680 = u8 2 items=["1", "2", "3"] ("axis")
                      w4681 = u8 1 items=["1", "2", "3"] ("axis")
                      w4690 = u8 0 items=["1", "2", "3"] ("axis")
                      w4679 = FALSE ("ANC connected")
                      n3938 = local read "Att DeviceHandle"() -> (w4692:u64)
                      n3939 = local read "Att Error"() -> (w4691:errorcluster)
                      n3940 = local read "ourDLL"() -> (w4678:path)
                      n3941 = call "ANC350v4_SetAxisOutput.vi"("deviceHandle"=w4692, "Path to *.DLL"=w4678, "axis"=w4690, "enable"=FALSE, "autoDisable"=TRUE, "error in"=w4691) -> ("deviceHandle"=w4684:u64, "error ANC350v4_setAxisOutput"=w4689:errorcluster)  [unwired: 7 in, 1 out]
                      n3942 = call "ANC350v4_SetAxisOutput.vi"("deviceHandle"=w4684, "Path to *.DLL"=w4678, "axis"=w4681, "enable"=FALSE, "autoDisable"=TRUE, "error in"=w4689) -> ("deviceHandle"=w4685:u64, "error ANC350v4_setAxisOutput"=w4688:errorcluster)  [unwired: 7 in, 1 out]
                      n3943 = call "ANC350v4_SetAxisOutput.vi"("deviceHandle"=w4685, "Path to *.DLL"=w4678, "axis"=w4680, "enable"=FALSE, "autoDisable"=TRUE, "error in"=w4688) -> ("deviceHandle"=w4686:u64, "error ANC350v4_setAxisOutput"=w4687:errorcluster)  [unwired: 7 in, 1 out]
                      n3944 = call "ANC350v4sub_Disconnect.vi"("ANC350v4_Handle"=w4686, "Path to *.DLL"=w4678, "error in"=w4687) -> ("error ANC350v4_Dis/Connect"=w4694:errorcluster)  [unwired: 12 in]
                      n3945 = local write "Voltage Output?"(w4679) -> ()
                      n3946 = local write "ANC connected"(w4679) -> ()
                      n3947 = local write "Att Error"(w4694) -> ()
                    }
                  }
                }
                frame #9 {
                  # "Montana Cryostation s50"
                  n3948 = local read "Cryostation On?"() -> (w4695:bool)
                  n3949 = case shown="True" w4695 {
                    frame False {
                    }
                    frame True {
                      n3950 = local read "Cryostation ID"() -> (w4696:refnum<k5>)
                      n3951 = call "CryoDisconnect.vi"("connection ID"=w4696) -> ()
                    }
                  }
                }
                frame #10 {
                  n3952 = local read "PicoHarp On?"() -> (w4697:bool)
                  n3953 = case shown="True" w4697 {
                    frame False {
                    }
                    frame True {
                      n3954 = local read "PH_Init_Data"() -> (w4700:T11)
                      n3955 = Unbundle By Name(w4700) -> ("Deviceindex"=w4699:i32)
                      n3956 = local write "Connected"(FALSE) -> ()
                      n3957 = call "PH_Close.vi"("devidx"=w4699) -> ()
                    }
                  }
                }
              }
            }
          }
        }
        frame #2 {
          # "Save log file & empty strings for next operation"
          n3958 = local read "Initialise all devices?"() -> (w4701:bool)
          n3959 = property on="Experiment Graph Controls" class="TabCtl (strict)"() -> ("Pages"=w4706:refnum<vi>[])  [unwired: 2 in, 2 out]
          n3960 = case shown="True" w4701 {
            frame False {
            }
            frame True {
              n3961 = stacked-sequence {
                frame #0 {
                  # "save log file"
                  n3962 = local read "Experiment Name"() -> (w4709:string)
                  n3963 = local read "Log file"() -> (w4710:string)
                  n3964 = call "CreatePath.vi"("filetype"=enum16{".h5", ".txt"}.".txt", "FileName"=w4709) -> ("File path"=w4707:path)
                  n3965 = Write to Text File(file (use dialog)=w4707, text=w4710) -> ()  [unwired: 2 in, 3 out]
                }
              }
            }
          }
          n3966 = Index Array(array=w4706, index=6) -> (element=w4704:refnum<vi>)
          n3967 = property class="Page"(reference=w4704, "PageVis"=TRUE ("Page Visible")) -> ()  [unwired: 1 in, 2 out]
          n3968 = property on="Experiment Graph Controls" class="TabCtl (strict)"("Value"=T25."Settings" ("Experiment Graph Controls")) -> ()  [unwired: 2 in, 2 out]
        }
      }
    }
  }
  n3969 = disable-structure shown="Enabled" {
    frame Disabled {
    }
    frame Enabled {
      w4719 = T29."Disabled and Grayed Out" ("Disabled")
      w4717 = FALSE ("Visible")
      w4715 = FALSE ("Pause XY Map")
      w4716 = FALSE
      w4714 = FALSE ("Visible")
      w4725 = TRUE
      w4738 = dbl[] []
      w4744 = TRUE ("Visible")
      # "Progress bars"
      # "XYZ objective piezos and shutter"
      # "connected through"
      # "XY Scanning measurements"
      # "Polarisation measurement"
      # "Spectrum Custom"
      # "Spectrum with APDs"
      # "Acquire controls"
      # "Save controls"
      # "CCD"
      # "MonochromatorS"
      # "Rotation stages PR50PP"
      # "Main"
      # "Photodiode PM16-120"
      # "Steering mirror FSM 300"
      # "Settings for instrumentation"
      # "Contrôle manip GH013"
      n3970 = property on="CCD 1D Spectrum Main Energy Scale" class="XYGraph (strict)"("Plot.Visible?"=FALSE ("Plot.Visible"), "Plot.Line Width"=u8 0) -> ()  [unwired: 2 in, 2 out]
      n3971 = disable-structure shown="Disabled" {
        frame Disabled {
          n3972 = call "Define Home.vi"() -> ()  [unwired: 10 in, 2 out]
          n3973 = call "Wait For Motion Done.vi"() -> ()  [unwired: 10 in, 2 out]
          n3974 = call "Motor On.vi"() -> ()  [unwired: 10 in, 2 out]
          n3975 = call "Motor Off.vi"() -> ()  [unwired: 10 in, 2 out]
          n3976 = call "Move To Position.vi"() -> ()  [unwired: 10 in, 2 out]
          n3977 = call "Home.vi"() -> ()  [unwired: 10 in, 2 out]
        }
        frame Enabled {
        }
      }
      n3978 = local write "Photodiode Status"(FALSE) -> ()
      n3979 = property on="Polarisation 1D Spectrum Energy Scale" class="XYGraph (strict)"("Plot.Visible?"=FALSE ("Plot.Visible"), "Plot.Line Width"=u8 0) -> ()  [unwired: 2 in, 2 out]
      n3980 = property on="Pause XY Map" class="Bool (strict)"("Visible"=w4716, "Value"=w4715) -> ()  [unwired: 2 in, 2 out]
      n3981 = property on="Stop XY Map" class="Bool (strict)"("Visible"=w4716, "Value"=w4715) -> ()  [unwired: 2 in, 2 out]
      n3982 = local write "BackgroundSpec"(i32[] []) -> ()
      n3983 = property on="Stop fPow" class="Bool (strict)"("Visible"=w4717) -> ()  [unwired: 2 in, 2 out]
      n3984 = property on="Pause fPow" class="Bool (strict)"("Visible"=w4717) -> ()  [unwired: 2 in, 2 out]
      n3985 = property on="Elapsed (s)" class="DigNum (strict)"("Visible"=w4714) -> ()  [unwired: 2 in, 2 out]
      n3986 = disable-structure shown="Disabled" {
        disable-tunnel: w4714 -> [w4791 _]
        frame Disabled {
          n3987 = property on="Scan Main Progess Bar" class="Slide (strict)"("Visible"=w4791) -> ()  [unwired: 2 in, 2 out]
        }
        frame Enabled {
        }
      }
      n3988 = property on="Save fPow" class="Bool (strict)"("Visible"=TRUE) -> ()  [unwired: 2 in, 2 out]
      n3989 = local write "DotNum"(0.0 ("DotNum")) -> ()
      n3990 = control-ref of="Acquire Contrast"() -> (w4721:refnum<vi>)
      n3991 = control-ref of="Save Contrast"() -> (w4720:refnum<vi>)
      n3992 = Bundle(w4738, w4738) -> (w4737:cluster{dbl[], dbl[]})  [unwired: 1 in]
      n3993 = property class="Bool (strict)"(reference=w4720, "DisabledEnum"=w4719) -> ()  [unwired: 1 in, 2 out]
      n3994 = Build Array(w4737, w4737) -> ()  [unwired: 1 out]
      n3995 = control-ref of="Scanning Mode"() -> (w4784:refnum<vi>)
      n3996 = control-ref of="Scan Fast Axis"() -> (w4785:refnum<vi>)
      n3997 = property class="Bool (strict)"(reference=w4721, "DisabledEnum"=w4719) -> ()  [unwired: 1 in, 2 out]
      n3998 = control-ref of="Scan X Num. Pts"() -> (w4781:refnum<vi>)
      n3999 = control-ref of="Spectrum End Wavelength (nm)"() -> (w4752:refnum<vi>)
      n4000 = control-ref of="Spectrum Step Wavelength (nm)"() -> (w4751:refnum<vi>)
      n4001 = control-ref of="Spectrum Start Wavelength (nm)"() -> (w4750:refnum<vi>)
      n4002 = control-ref of="Spectrum Custom Mode"() -> (w4749:refnum<vi>)
      n4003 = control-ref of="Scan Y Center (V)"() -> (w4780:refnum<vi>)
      n4004 = control-ref of="Scan X Center (V)"() -> (w4783:refnum<vi>)
      n4005 = control-ref of="Scan Y Tot. Length"() -> (w4746:refnum<vi>)
      n4006 = control-ref of="Scan Y Res. (V)"() -> (w4779:refnum<vi>)
      n4007 = control-ref of="Scan X Tot. Length (V)"() -> (w4747:refnum<vi>)
      n4008 = control-ref of="Scan Y Num. Pts"() -> (w4778:refnum<vi>)
      n4009 = property on="StopPolar" class="Bool (strict)"("Visible"=w4744) -> ()  [unwired: 2 in, 2 out]
      n4010 = property on="PausePolar" class="Bool (strict)"("Visible"=w4744) -> ()  [unwired: 2 in, 2 out]
      n4011 = control-ref of="Scan X Res. (V)"() -> (w4782:refnum<vi>)
      n4012 = control-ref of="Polar Start Angle (°)"() -> (w4776:refnum<vi>)
      n4013 = control-ref of="Polar Step Angle (°)"() -> (w4774:refnum<vi>)
      n4014 = control-ref of="Polar End Angle (°)"() -> (w4775:refnum<vi>)
      n4015 = Build Array(w4752, w4751, w4750, w4749) -> (→"Scan Spectrum Cust Params":refnum<vi>[])
      n4016 = Build Array(w4785, w4784, w4783, w4782, w4781, w4780, w4779, w4778, w4747, w4746) -> (→"Scan XY Map Params":refnum<vi>[])
      n4017 = control-ref of="Save Polarisation"() -> (w4741:refnum<vi>)
      n4018 = property on="Acquire XY Map" class="Bool (strict)"("Visible"=w4725, "Value"=FALSE ("Acquire XY Map")) -> ()  [unwired: 2 in, 2 out]
      n4019 = property on="Save XY Map" class="Bool (strict)"("Visible"=w4725) -> ()  [unwired: 2 in, 2 out]
      n4020 = control-ref of="Acquire Polarisation"() -> (w4742:refnum<vi>)
      n4021 = control-ref of="Polar mode"() -> (w4773:refnum<vi>)
      n4022 = Build Array(w4773, w4776, w4775, w4774) -> (w4743:refnum<vi>[])
      "Scan Polar Params" <- w4743
      n4023 = Build Array (concatenate)(w4743, w4742, w4741) -> (→"Scan Polar AllParams":refnum<vi>[])
      n4024 = control-ref of="LinTFine Start Pos (usteps)"() -> (w4770:refnum<vi>)
      n4025 = control-ref of="LinTFines Step Pos (usteps)"() -> (w4769:refnum<vi>)
      n4026 = control-ref of="LinTFine End Pos (usteps)"() -> (w4768:refnum<vi>)
      n4027 = control-ref of="Acquire Contrast"() -> (w4759:refnum<vi>)
      n4028 = property on="Background substract" class="Enum (strict)"("Value"=enum16{"None", "Shutter"}."None" ("Background substract")) -> ()  [unwired: 2 in, 2 out]
      n4029 = control-ref of="Save Michelson"() -> (w4754:refnum<vi>)
      n4030 = control-ref of="Acquire Michelson"() -> (w4755:refnum<vi>)
      n4031 = control-ref of="LinT Step Pos (mm)"() -> (w4757:refnum<vi>)
      n4032 = control-ref of="LinT Start Pos (mm)"() -> (w4758:refnum<vi>)
      n4033 = control-ref of="LinT End pos (mm)"() -> (w4756:refnum<vi>)
      n4034 = control-ref of="Stop Spectrum Custom"() -> ()  [unwired: 1 out]
      n4035 = local write "Background taken?"(FALSE ("Background taken?")) -> ()
      n4036 = control-ref of="Stop Contrast"() -> (w4772:refnum<vi>)
      n4037 = control-ref of="Pause Contrast"() -> (w4771:refnum<vi>)
      n4038 = Build Array(w4758, w4757, w4756, w4770, w4769, w4768) -> (→"Scan Contrast Ctrls":refnum<vi>[])
      n4039 = Bundle("LinTFine Start Pos (usteps)"=w4770, "LinTFines Step Pos (usteps)"=w4769, "LinTFine End Pos (usteps)"=w4768, "Acquire Contrast"=w4759, "Stop Contrast"=w4772, "Pause Contrast"=w4771) -> ()  [unwired: 1 in, 1 out]
      n4040 = control-ref of="Scan Contrast Ctrls"() -> ()  [unwired: 1 out]
      n4041 = Bundle("LinT Start Pos (mm)"="LinT Start Pos (mm)", "LinT Step Pos (mm)"="LinT Step Pos (mm)", "LinT End pos (mm)"="LinT End pos (mm)", "LinTFine Start Pos (usteps)"="LinTFine Start Pos (usteps)", "LinTFines Step Pos (usteps)"="LinTFines Step Pos (usteps)", "LinTFine End Pos (usteps)"="LinTFine End Pos (usteps)") -> (→"Scan Translation Params":T27)  [unwired: 1 in]
      n4042 = Build Array(w4758, w4757, w4756, w4755, w4754) -> (→"Scan Translation Coarse Ctrls":refnum<vi>[])
      n4043 = disable-structure shown="Enabled" {
        frame Enabled {
          # "Documentation Buttons"
        }
        frame Disabled {
        }
      }
      n4044 = control-ref of="MasterStop"() -> (w4729:refnum<vi>)
      n4045 = control-ref of="MasterPause"() -> (w4730:refnum<vi>)
      n4046 = property on="Elapsed (s)" class="DigNum (strict)"("Visible"=FALSE) -> ()  [unwired: 2 in, 2 out]
      n4047 = control-ref of="ExperimentStopped?"() -> (w4728:refnum<vi>)
      n4048 = call "CheckStopAndReset.vi"("ExperimentStopped?"=w4728, "MasterStop"=w4729, "MasterPause"=w4730) -> ()
      n4049 = control-ref of="Mono2 Wavelength (nm)"() -> ()  [unwired: 1 out]
      n4050 = control-ref of="MasterStop"() -> ()  [unwired: 1 out]
      n4051 = control-ref of="MasterPause"() -> ()  [unwired: 1 out]
      n4052 = control-ref of="Pause fPow"() -> ()  [unwired: 1 out]
      n4053 = control-ref of="Save PLE"() -> (w4735:refnum<vi>)
      n4054 = control-ref of="PLE Start (nm)"() -> (w4731:refnum<vi>)
      n4055 = control-ref of="PLE End (nm)"() -> (w4732:refnum<vi>)
      n4056 = control-ref of="PLE Step (nm)"() -> (w4733:refnum<vi>)
      n4057 = control-ref of="Acquire PLE"() -> (w4734:refnum<vi>)
      n4058 = property on="HR mode" class="Ring (strict)"("DisabledEnum"=T29."Disabled and Grayed Out" ("Disabled")) -> ()  [unwired: 2 in, 2 out]
      n4059 = Build Array(w4734, w4735, w4731, w4732, w4733) -> (→"Scan PLE AllParams":refnum<vi>[])
      "ESP300 COM Port" <- refnum<visa-resource-name> "COM4" ("ESP300 COM Port")
      "PD 1D Spectrum" <- dbl[][] []
      "Background taken?" <- FALSE ("Background taken?")
    }
  }
